vi "TLB Native Dynamic Events ver 0.26b.vi"() -> ()   [LabVIEW 2018] (continued)
      tunnel: [w2960 w2972 w2987 w3011 w3021 w3036 w3050 w3065 w3080 w3095 w3109 w3121 w3137 w3149 w3171 w3194 w3211 w3220 w3237 w3263 w3274 w3287 w3302 w3315 w3330 w3351 w3387 w3417 w3429 w3442 w3454 w3470 w3486 w3499 w3510 w3537 w3560 w3572 w3580 w3591 w3602 w3615 w3628 w3647 w3658 w3675 w3682 w3703 w3718 w3733 w3748 w3763 w3778 w3792] -> w237
      tunnel: w235 -> [w2958 w2971 w2988 w3012 w3022 w3037 w3051 w3064 w3081 w3096 w3108 w3120 w3136 w3148 w3168 w3195 w3212 w3219 w3234 w3260 w3273 w3286 w3301 w3314 w3329 w3349 w3385 w3415 w3428 w3441 w3453 w3469 w3485 w3498 w3509 w3538 w3561 w3573 w3579 w3590 w3601 w3614 w3627 w3648 w3659 w3676 w3681 w3697 w3712 w3727 w3742 w3757 w3772 w3786]
      tunnel: [w2958 w2971 w2988 w3012 w3022 w3037 w3051 w3064 w3081 w3096 w3108 w3120 w3136 w3148 w3168 w3195 w3212 w3219 w3234 w3260 w3273 w3286 w3301 w3314 w3328 w3348 w3384 w3415 w3428 w3441 w3453 w3469 w3485 w3498 w3509 w3538 w3561 w3573 w3579 w3590 w3601 w3614 w3627 w3648 w3659 w3676 w3681 w3697 w3710 w3725 w3740 w3755 w3770 w3785] -> w234
      tunnel: w232 -> [_ _ _ _ _ _ _ _ _ _ _ _ _ _ _ _ _ _ _ _ _ _ _ _ _ _ _ _ _ _ _ _ _ _ _ _ _ _ _ _ _ _ _ _ _ w3667 _ _ _ _ _ _ _ _]
      tunnel: [w2957 w2970 w2982 w3002 w3016 w3031 w3046 w3060 w3076 w3090 w3105 w3119 w3130 w3147 w3165 w3186 w3213 w3218 w3231 w3259 w3272 w3285 w3300 w3311 w3322 w3342 w3376 w3414 w3427 w3440 w3458 w3463 w3479 w3495 w3507 w3522 w3554 w3565 w3585 w3589 w3600 w3613 w3626 w3639 w3660 w3665 w3680 w3696 w3707 w3722 w3737 w3752 w3767 w3782] -> w228
      tunnel: w229 -> [w2957 w2970 w2982 w3002 w3016 w3031 w3046 w3060 w3076 w3090 w3105 w3119 w3130 w3147 w3165 w3187 w3213 w3218 w3231 w3259 w3272 w3285 w3300 w3311 w3322 w3343 w3377 w3414 w3427 w3440 w3458 w3463 w3479 w3495 w3507 w3522 w3554 w3565 w3585 w3589 w3600 w3613 w3626 w3639 w3660 w3665 w3680 w3696 w3707 w3722 w3737 w3752 w3767 w3782]
      tunnel: w226 -> [_ _ _ _ _ _ _ _ w3075 _ _ _ _ _ _ _ _ _ _ _ _ _ _ _ _ _ _ _ _ _ _ _ _ _ _ _ _ _ _ _ _ _ _ _ _ _ _ _ _ _ _ _ _ _]
      tunnel: w224 -> [w2956 w2969 w2981 w2996 w3015 w3030 w3045 w3059 w3073 w3089 w3104 w3118 w3129 w3146 w3164 w3182 w3206 w3217 w3229 w3258 w3271 w3284 w3299 w3310 w3325 w3345 w3380 w3413 w3426 w3439 w3450 w3462 w3478 w3494 w3506 w3519 w3553 w3564 w3576 w3588 w3599 w3612 w3625 w3638 w3651 w3664 w3679 w3695 w3706 w3721 w3736 w3751 w3766 w3781]
      tunnel: [w2956 w2969 w2981 w2996 w3015 w3030 w3045 w3059 w3073 w3089 w3104 w3118 w3129 w3146 w3164 w3182 w3205 w3217 w3229 w3258 w3271 w3284 w3299 w3310 w3324 w3344 w3379 w3413 w3426 w3439 w3450 w3462 w3478 w3494 w3506 w3519 w3553 w3564 w3576 w3588 w3599 w3612 w3625 w3638 w3651 w3664 w3679 w3695 w3706 w3721 w3736 w3751 w3766 w3781] -> w223
      tunnel: [_ _ _ _ _ _ _ _ _ _ _ _ _ _ _ _ _ _ _ _ _ _ _ _ _ _ _ _ _ _ _ _ _ _ _ w3518 w3548 _ _ _ _ _ _ _ _ _ _ _ _ _ _ _ _ _] -> w221
      tunnel: w219 -> [w2955 w2968 w2980 w2995 w3014 w3029 w3044 w3058 w3072 w3088 w3103 w3117 w3128 w3145 w3163 w3181 w3197 w3216 w3227 w3257 w3270 w3283 w3298 w3309 w3326 w3346 w3381 w3412 w3425 w3438 w3449 w3461 w3477 w3493 w3505 w3517 w3552 w3563 w3575 w3587 w3598 w3611 w3624 w3637 w3650 w3663 w3678 w3694 w3705 w3720 w3735 w3750 w3765 w3780]
      tunnel: [w2955 w2968 w2980 w2995 w3014 w3029 w3044 w3058 w3072 w3088 w3103 w3117 w3128 w3145 w3163 w3181 w3197 w3216 w3227 w3257 w3270 w3283 w3298 w3309 w3326 w3346 w3381 w3412 w3425 w3438 w3449 w3461 w3477 w3493 w3505 w3517 w3552 w3563 w3575 w3587 w3598 w3611 w3624 w3637 w3650 w3663 w3678 w3694 w3705 w3720 w3735 w3750 w3765 w3780] -> w218
      tunnel: w214 -> [w2954 w2967 w2979 w2994 w3013 w3028 w3043 w3057 w3071 w3087 w3102 w3116 w3127 w3144 w3162 w3178 w3196 w3215 w3226 w3256 w3269 w3282 w3297 w3308 w3321 w3339 w3374 w3411 w3424 w3437 w3448 w3460 w3476 w3492 w3504 w3516 w3546 w3562 w3574 w3586 w3597 w3610 w3623 w3636 w3649 w3662 w3677 w3693 w3704 w3719 w3734 w3749 w3764 w3779]
      tunnel: [w2954 w2967 w2979 w2994 w3013 w3028 w3043 w3057 w3071 w3087 w3102 w3116 w3127 w3144 w3162 w3178 w3196 w3215 w3226 w3256 w3269 w3282 w3297 w3308 w3321 w3339 w3374 w3411 w3424 w3437 w3448 w3460 w3476 w3492 w3504 w3516 w3539 w3562 w3574 w3586 w3597 w3610 w3623 w3636 w3649 w3662 w3677 w3693 w3704 w3719 w3734 w3749 w3764 w3779] -> w213
      frame "Exit" {
        # ">>State Logic  >>"
        # ">>> Time cluster >>>"
        # ">>> Yaw >>>"
        # ">>> Stepper position >>>"
        # ">>> Encoders >>>"
        # ">>> Object detection >>>"
        # ">>> Ultrasonic Sensors Detect >>>"
        n70 = call "Imaq Dispose"("All Images? (No)"=TRUE) -> ()  [unwired: 5 in, 1 out]
      }
      frame "----Movement States----" {
        # ">>State Logic  >>"
        # ">>> Time cluster >>>"
        # ">>> Yaw >>>"
        # ">>> Stepper position >>>"
        # ">>> Encoders >>>"
        # ">>> Object detection >>>"
        # ">>> Ultrasonic Sensors Detect >>>"
      }
      frame "FORWARD" {
        # ">>State Logic  >>"
        # ">>> Time cluster >>>"
        # ">>> Yaw >>>"
        # ">>> Stepper position >>>"
        # ">>> Encoders >>>"
        # ">>> Object detection >>>"
        # ">>> Ultrasonic Sensors Detect >>>"
        n71 = Unbundle By Name(w2987) -> ("Yaw"=w2983:dbl)
        n72 = call "MOTOR CONTROL WITH PID AE.vi"("Yaw"=w2983, "Speed"=50.0, "Direction"=MOTOR_CONTROL_WITH_PID_AE_DIRECTION_TYPE_DEF."y-axis movement", "AE Mode"=MOTOR_CONTROL_WITH_PID_AE_DATA_MODE_TYPE_DEF."Write to AE") -> ()  [unwired: 1 out]
      }
      frame "FORWARD - IR ASSIST" {
        # ">>State Logic  >>"
        # ">>> Time cluster >>>"
        # ">>> Yaw >>>"
        # ">>> Stepper position >>>"
        # ">>> Encoders >>>"
        # ">>> Object detection >>>"
        # ">>> Ultrasonic Sensors Detect >>>"
        n73 = Unbundle By Name(w3002) -> ("Left IR Sensor"=w3001:dbl)
        n74 = Subtract(x=w3001, y=10.0) -> (x-y=w2999:dbl)
        n75 = Multiply(x=w2999, y=0.2) -> (x*y=w2997:dbl)
        n76 = call "MOTOR CONTROL WITH PID AE.vi"("Yaw"=w2997, "Speed"=40.0, "Direction"=MOTOR_CONTROL_WITH_PID_AE_DIRECTION_TYPE_DEF."y-axis movement", "AE Mode"=MOTOR_CONTROL_WITH_PID_AE_DATA_MODE_TYPE_DEF."Write to AE") -> ()  [unwired: 1 out]
      }
      frame "LEFT" {
        # ">>State Logic  >>"
        # ">>> Time cluster >>>"
        # ">>> Yaw >>>"
        # ">>> Stepper position >>>"
        # ">>> Encoders >>>"
        # ">>> Object detection >>>"
        # ">>> Ultrasonic Sensors Detect >>>"
        n77 = Unbundle By Name(w3021) -> ("Yaw"=w3018:dbl)
        n78 = call "MOTOR CONTROL WITH PID AE.vi"("Yaw"=w3018, "Speed"=-20.0, "Direction"=MOTOR_CONTROL_WITH_PID_AE_DIRECTION_TYPE_DEF."x-axis movement", "AE Mode"=MOTOR_CONTROL_WITH_PID_AE_DATA_MODE_TYPE_DEF."Write to AE") -> ()  [unwired: 1 out]
      }
      frame "RIGHT" {
        # ">>> Time cluster >>>"
        # ">>> Yaw >>>"
        # ">>> Stepper position >>>"
        # ">>> Encoders >>>"
        # ">>> Object detection >>>"
        # ">>> Ultrasonic Sensors Detect >>>"
        n79 = Unbundle By Name(w3036) -> ("Yaw"=w3032:dbl)
        n80 = call "MOTOR CONTROL WITH PID AE.vi"("Yaw"=w3032, "Speed"=20.0, "Direction"=MOTOR_CONTROL_WITH_PID_AE_DIRECTION_TYPE_DEF."x-axis movement", "AE Mode"=MOTOR_CONTROL_WITH_PID_AE_DATA_MODE_TYPE_DEF."Write to AE") -> ()  [unwired: 1 out]
      }
      frame "R-ACW" {
        # ">>> IR Sensors >>>"
        # ">>> Time cluster >>>"
        # ">>> Yaw >>>"
        # ">>> Stepper position >>>"
        # ">>> Encoders >>>"
        # ">>> Object detection >>>"
        # ">>> Ultrasonic Sensors Detect >>>"
        n81 = call "MOTOR CONTROL WITH PID AE.vi"("Speed"=10.0, "Direction"=MOTOR_CONTROL_WITH_PID_AE_DIRECTION_TYPE_DEF."rotation", "AE Mode"=MOTOR_CONTROL_WITH_PID_AE_DATA_MODE_TYPE_DEF."Write to AE") -> ()  [unwired: 1 in, 1 out]
      }
      frame "R-CW" {
        (unwired) -0.2 ("Speed")
        # ">>> Time cluster >>>"
        # ">>> Yaw >>>"
        # ">>> Stepper position >>>"
        # ">>> Encoders >>>"
        # ">>> Object detection >>>"
        # ">>> Ultrasonic Sensors Detect >>>"
        n82 = call "MOTOR CONTROL WITH PID AE.vi"("Speed"=-10.0, "Direction"=MOTOR_CONTROL_WITH_PID_AE_DIRECTION_TYPE_DEF."rotation", "AE Mode"=MOTOR_CONTROL_WITH_PID_AE_DATA_MODE_TYPE_DEF."Write to AE") -> ()  [unwired: 1 in, 1 out]
      }
      frame "X AXIS - SLOW" {
        # ">>> Line Sensor Cluster>>>"
        # ">>> IR Sensors >>>"
        # ">>> Time cluster >>>"
        # ">>> Yaw >>>"
        # ">>> Stepper position >>>"
        # ">>> Encoders >>>"
        # ">>> Object detection >>>"
        # ">>> Ultrasonic Sensors Detect >>>"
        n83 = Unbundle By Name(w3075) -> ("xSpeed"=w3074:dbl)
        n84 = Unbundle By Name(w3080) -> ("Yaw"=w3077:dbl)
        n85 = call "MOTOR CONTROL WITH PID AE.vi"("Yaw"=w3077, "Speed"=w3074, "Direction"=MOTOR_CONTROL_WITH_PID_AE_DIRECTION_TYPE_DEF."x-axis movement", "AE Mode"=MOTOR_CONTROL_WITH_PID_AE_DATA_MODE_TYPE_DEF."Write to AE") -> ()  [unwired: 1 out]
      }
      frame "REVERSE" {
        # ">>> Time cluster >>>"
        # ">>> Yaw >>>"
        # ">>> Stepper position >>>"
        # ">>> Encoders >>>"
        # ">>> Object detection >>>"
        # ">>> Ultrasonic Sensors Detect >>>"
        n86 = Unbundle By Name(w3095) -> ("Yaw"=w3091:dbl)
        n87 = call "MOTOR CONTROL WITH PID AE.vi"("Yaw"=w3091, "Speed"=-50.0, "Direction"=MOTOR_CONTROL_WITH_PID_AE_DIRECTION_TYPE_DEF."y-axis movement", "AE Mode"=MOTOR_CONTROL_WITH_PID_AE_DATA_MODE_TYPE_DEF."Write to AE") -> ()  [unwired: 1 out]
      }
      frame "STOP" {
        n88 = Wait (ms)(milliseconds to wait=u32 100) -> ()  [unwired: 1 out]
        n89 = call "MOTOR CONTROL WITH PID AE.vi"("Direction"=MOTOR_CONTROL_WITH_PID_AE_DIRECTION_TYPE_DEF."stop", "AE Mode"=MOTOR_CONTROL_WITH_PID_AE_DATA_MODE_TYPE_DEF."Write to AE") -> ()  [unwired: 2 in, 1 out]
      }
      frame "----SENSOR READING---- " {
      }
      frame "READ ENCODERS" {
        # ">>> Time cluster >>>"
        # ">>> Yaw >>>"
        # ">>> Stepper position >>>"
        # ">>> Object detection >>>"
        # ">>> Current encoder distance >>>"
        # ">>> Ultrasonic Sensors Detect >>>"
        n90 = call "MOTOR CONTROL WITH PID AE.vi"("AE Mode"=MOTOR_CONTROL_WITH_PID_AE_DATA_MODE_TYPE_DEF."Read from AE") -> ("Speed & distance"=w3134:T15)  [unwired: 3 in]
        n91 = Unbundle By Name(w3134) -> ("xDistance"=w3133:dbl, "yDistance"=w3132:dbl, "wDistance"=w3131:dbl)
        n92 = Bundle By Name(cluster=w3141, "xDistance"=w3133, "yDistance"=w3132, "wDistance"=w3131) -> (w3140:T8)
      }
      frame "READ ULTRASONIC" {
        (unwired) navX_type_def."Read Values" ("Mode")
        (unwired) MOTOR_CONTROL_NO_PID_Type_Def."Latch" ("Direction")
        # ">>> Line Sensor Cluster>>>"
        # ">>> IR Sensors >>>"
        # ">>State Logic  >>"
        # ">>> Time cluster >>>"
        # ">>> Ultrasonic Sensors Detect >>>"
        # ">>> Object detection >>>"
        # ">>> Encoders >>>"
        # ">>> Stepper position >>>"
        # ">>> Yaw >>>"
        n93 = call "Arduino Interfacing VI.vi"("AE Mode"=Arduino_Interfacing."Read From Arduino") -> ("Arduino Data"=w3154:T17)  [unwired: 3 in, 1 out]
        n94 = Unbundle By Name(w3154) -> ("PING A"=w3153:u8, "PING B"=w3152:u8, "PING C"=w3151:u8, "PING D"=w3150:u8)
        n95 = Bundle By Name(cluster=w3160, "PING_A"=w3153, "PING_B"=w3152, "PING_C"=w3151, "PING_D"=w3150) -> (w3161:T9)
      }
      frame "READ NAVX" {
        # ">> Item Selection Bias >>"
        # ">>State Logic  >>"
        # ">>> Line Sensor Cluster>>>"
        # ">>> IR Sensors >>>"
        # ">>> Time cluster >>>"
        # ">>> Yaw >>>"
        # ">>> Ultrasonic Sensors Detect >>>"
        # ">>> Object detection >>>"
        # ">>> Encoders >>>"
        # ">>> Stepper position >>>"
        n96 = call "navX reading VI.vi"("Mode"=navX_type_def."Read Values") -> ("NavX Readings"=w3167:T16)  [unwired: 2 in, 3 out]
        n97 = Unbundle By Name(w3167) -> ("Heading"=w3166:dbl)
        n98 = Unbundle By Name(w3167) -> ("Yaw"=w3170:dbl)
        n99 = Bundle By Name(cluster=w3172, "Yaw"=w3170, "Compass"=w3166) -> (w3171:T6)
      }
      frame "READ IR" {
        w3180 = T42 [enum."B/AI2"] items=["Not Connected", "AudioIn/Left", "AudioIn/Right", "C/AI0", "C/AI1", "A/AI0", "A/AI1", "A/AI2", "A/AI3", "A/AI4", "A/AI5", "A/AI6", "A/AI7", "B/AI0", "B/AI1", "B/AI2", "B/AI3", "B/AI4", "B/AI5", "B/AI6", "B/AI7", "AI/AI0", "AI/AI1", "AI/AI2", "AI/AI3", "A/AI0 (DIFF)", "A/AI1 (DIFF)", "A/AI2 (DIFF)", "A/AI3 (DIFF)", "B/AI0 (DIFF)", "B/AI1 (DIFF)", "B/AI2 (DIFF)", "B/AI3 (DIFF)"] ("AI Channel")
        w3184 = T42 [enum."B/AI1"] items=["Not Connected", "AudioIn/Left", "AudioIn/Right", "C/AI0", "C/AI1", "A/AI0", "A/AI1", "A/AI2", "A/AI3", "A/AI4", "A/AI5", "A/AI6", "A/AI7", "B/AI0", "B/AI1", "B/AI2", "B/AI3", "B/AI4", "B/AI5", "B/AI6", "B/AI7", "AI/AI0", "AI/AI1", "AI/AI2", "AI/AI3", "A/AI0 (DIFF)", "A/AI1 (DIFF)", "A/AI2 (DIFF)", "A/AI3 (DIFF)", "B/AI0 (DIFF)", "B/AI1 (DIFF)", "B/AI2 (DIFF)", "B/AI3 (DIFF)"] ("AI Channel")
        w3189 = T42 [enum."B/AI0"] items=["Not Connected", "AudioIn/Left", "AudioIn/Right", "C/AI0", "C/AI1", "A/AI0", "A/AI1", "A/AI2", "A/AI3", "A/AI4", "A/AI5", "A/AI6", "A/AI7", "B/AI0", "B/AI1", "B/AI2", "B/AI3", "B/AI4", "B/AI5", "B/AI6", "B/AI7", "AI/AI0", "AI/AI1", "AI/AI2", "AI/AI3", "A/AI0 (DIFF)", "A/AI1 (DIFF)", "A/AI2 (DIFF)", "A/AI3 (DIFF)", "B/AI0 (DIFF)", "B/AI1 (DIFF)", "B/AI2 (DIFF)", "B/AI3 (DIFF)"] ("AI Channel")
        # ">>> Line Sensor Cluster>>>"
        # ">>> IR Sensors >>>"
        # ">>State Logic  >>"
        # ">>> Time cluster >>>"
        # ">>> Ultrasonic Sensors Detect >>>"
        # ">>> Object detection >>>"
        # ">>> Encoders >>>"
        # ">>> Stepper position >>>"
        # ">>> Yaw >>>"
        n100 = call <vilib>:"Sharp IR.vi"("AI Channel"=w3189) -> ("Sharp IR Distance"=w3185:dbl)  [unwired: 8 in, 2 out]
        n101 = call <vilib>:"Sharp IR.vi"("AI Channel"=w3184) -> ("Sharp IR Distance"=w3183:dbl)  [unwired: 8 in, 2 out]
        n102 = call <vilib>:"Sharp IR.vi"("AI Channel"=w3180) -> ("Sharp IR Distance"=w3179:dbl)  [unwired: 8 in, 2 out]
        n103 = Bundle By Name(cluster=w3187, "Left IR Sensor"=w3185, "Arm IR Sensor"=w3183, "Bottom IR Sensor"=w3179) -> (w3186:T5)
      }
      frame "READ LINE SENSOR" {
        # ">>> IR Sensors >>>"
        # ">>> Line Sensor Cluster>>>"
        # ">>State Logic  >>"
        # ">>> Time cluster >>>"
        # ">>> Object detection >>>"
        # ">>> Yaw >>>"
        # ">>> Ultrasonic Sensors Detect >>>"
        # ">>> Encoders >>>"
        # ">>> Stepper position >>>"
        n104 = call "Line Sensor AE.vi"("AE State"=Line_Sensor_AE_Type_Def."READ FROM LINE SENSORS") -> ("Line Detected?"=w3203:bool, "Line Sensor Raw Values"=w3202:T44)
        n105 = Unbundle By Name(w3202) -> ("S1"=w3201:dbl, "S2"=w3200:dbl, "S3"=w3199:dbl, "S4"=w3198:dbl)
        n106 = Bundle By Name(cluster=w3206, "Line Detected?"=w3203, "S1"=w3201, "S2"=w3200, "S3"=w3199, "S4"=w3198) -> (w3205:T4)
      }
      frame "----SYSTEM MODES----" {
        (unwired) I2C_MASTER_Type_Def."Last State" ("Arduino Mode")
        # ">>> Object detection >>>"
        # ">>> Yaw >>>"
        # ">>> Ultrasonic Sensors Detect >>>"
        # ">>> Encoders >>>"
        # ">>> Stepper position >>>"
      }
      frame "INIT" {
        w3249 = u8 0
        w3250 = 0.0
        # ">>> IR Sensors >>>"
        # ">>> IR Sensors >>>"
        # ">>> Line Sensor Cluster>>>"
        # ">>> Time cluster >>>"
        # ">>> Object detection >>>"
        # ">>> Yaw >>>"
        # ">>> Ultrasonic Sensors Detect >>>"
        # ">>> Encoders >>>"
        # ">>> Stepper position >>>"
        # ">>State Logic  >>"
        n107 = call "Arduino Interfacing VI.vi"("AE Mode"=Arduino_Interfacing."Initialize") -> ()  [unwired: 3 in, 2 out]
        n108 = call "FGV Stop.vi"("Init/Read/Write State"=States_for_Action_Engine."Initialize") -> ()  [unwired: 2 in, 2 out]
        n109 = call "Elasped Timer.vi"("Action"=Elapsed_timer_control."Initialize") -> ()  [unwired: 7 in, 4 out]
        n110 = call "MOTOR CONTROL WITH PID AE.vi"("AE Mode"=MOTOR_CONTROL_WITH_PID_AE_DATA_MODE_TYPE_DEF."Init AE") -> ()  [unwired: 3 in, 1 out]
        n111 = call "IMAQ Reference AE.vi"("IMAQ AE States"=IMAQ_Reference_AE."Initialize AE") -> ()  [unwired: 1 in, 2 out]
        n112 = call "Line Sensor AE.vi"("AE State"=Line_Sensor_AE_Type_Def."INIT AE") -> ()  [unwired: 2 out]
        n113 = Bundle By Name(cluster=w3243, "Recognized Object"=FALSE, "Object X coordinate"=0.0, "Object Y coordinate"=0.0) -> (w3242:T11)
        n114 = Bundle By Name(cluster=w3248, "y Stepper Position"=u8 0, "z Stepper Position"=u8 0) -> (w3247:T7)
        n115 = Bundle By Name(cluster=w3252, "xDistance"=w3250, "yDistance"=w3250, "wDistance"=w3250) -> (w3251:T8)
        n116 = Bundle By Name(cluster=w3254, "PING_A"=w3249, "PING_B"=w3249, "PING_C"=w3249, "PING_D"=w3249) -> (w3255:T9)
        n117 = Bundle By Name(cluster=w3238, "Yaw"=0.0) -> (w3237:T6)
      }
      frame "ARDUINO - ULTRASONIC" {
        # ">>> Time cluster >>>"
        # ">>> Line Sensor Cluster>>>"
        # ">>> Object detection >>>"
        # ">>> Yaw >>>"
        # ">>> Ultrasonic Sensors Detect >>>"
        # ">>> Encoders >>>"
        # ">>> Stepper position >>>"
        # ">>State Logic  >>"
        n118 = call "Arduino Interfacing VI.vi"("Data to Write"=I2C_MASTER_WRITE_NEW_Type_Def."Ultrasonic sensors", "AE Mode"=Arduino_Interfacing."Write to Arduino") -> ()  [unwired: 2 in, 2 out]
      }
      frame "NAVX CALIBRATE" {
        # ">>> Object detection >>>"
        # ">>> Yaw >>>"
        # ">>> Ultrasonic Sensors Detect >>>"
        # ">>> Encoders >>>"
        # ">>> Stepper position >>>"
        # ">>State Logic  >>"
        # "Adds a 15 second delay to the startup process \nfor the NavX to calibrate"
        n119 = Wait (ms)(milliseconds to wait=u32 1000) -> ()  [unwired: 1 out]
      }
      frame "NO ACTION", Default {
        (unwired) u8 0 ("y Stepper value")
        (unwired) TRUE ("Latch")
        (unwired) navX_type_def."Read Values" ("Mode")
        (unwired) MOTOR_CONTROL_NO_PID_Type_Def."Latch" ("Direction")
        # ">>> Object detection >>>"
        # ">>> Yaw >>>"
        # ">>> Ultrasonic Sensors Detect >>>"
        # ">>> Encoders >>>"
        # ">>> Stepper position >>>"
        # ">>State Logic  >>"
        n120 = case shown="4" w3291 {
          tunnel: [0 100] -> w3293
          frame 1, Default {
          }
          frame 4 {
          }
        }
      }
      frame "----RESET CASES----" {
        (unwired) I2C_MASTER_Type_Def."Last State" ("Arduino Mode")
        # ">>> Object detection >>>"
        # ">>> Yaw >>>"
        # ">>> Ultrasonic Sensors Detect >>>"
        # ">>> Encoders >>>"
        # ">>> Stepper position >>>"
        # ">>State Logic  >>"
      }
      frame "RESET ENCODERS" {
        # ">>> Object detection >>>"
        # ">>> Yaw >>>"
        # ">>> Ultrasonic Sensors Detect >>>"
        # ">>> Encoders >>>"
        # ">>> Stepper position >>>"
        # ">>State Logic  >>"
        n121 = call "MOTOR CONTROL WITH PID AE.vi"("Direction"=MOTOR_CONTROL_WITH_PID_AE_DIRECTION_TYPE_DEF."reset encoders", "AE Mode"=MOTOR_CONTROL_WITH_PID_AE_DATA_MODE_TYPE_DEF."Write to AE") -> ()  [unwired: 2 in, 1 out]
      }
      frame "RESET FLAGS" {
        # ">>> Line Sensor Cluster>>>"
        # ">>> IR Sensors >>>"
        # ">>> Time cluster >>>"
        # ">>> Object detection >>>"
        # ">>> Yaw >>>"
        # ">>> Ultrasonic Sensors Detect >>>"
        # ">>> Encoders >>>"
        # ">>> Stepper position >>>"
        # ">>> Line Sensor Cluster>>>"
        # ">>> IR Sensors >>>"
        # ">>> Time cluster >>>"
        # ">>> Object detection >>>"
        # ">>> Yaw >>>"
        # ">>> Ultrasonic Sensors Detect >>>"
        # ">>> Encoders >>>"
        # ">>> Stepper position >>>"
        # "Resets BOOLEAN FLAGS only"
        n122 = Wait (ms)(milliseconds to wait=u32 20) -> ()  [unwired: 1 out]
        n123 = Bundle By Name(cluster=w3335, "Recognized Object"=FALSE) -> (w3334:T11)
        n124 = Bundle By Name(cluster=w3325, "Line Detected?"=FALSE) -> (w3324:T4)
        n125 = Bundle By Name(cluster=w3329, "Time up flag"=FALSE) -> (w3328:T3)
      }
      frame "RESET SENSOR VALUES" {
        w3340 = 0.0 ("S4")
        w3341 = 0.0 ("S4")
        # "Resets SENSOR VALUES only"
        # ">>> Line Sensor Cluster>>>"
        # ">>> IR Sensors >>>"
        # ">>> Time cluster >>>"
        # ">>> Object detection >>>"
        # ">>> Yaw >>>"
        # ">>> Ultrasonic Sensors Detect >>>"
        # ">>> Encoders >>>"
        # ">>> Stepper position >>>"
        # ">>> Line Sensor Cluster>>>"
        # ">>> IR Sensors >>>"
        # ">>> Time cluster >>>"
        # ">>> Object detection >>>"
        # ">>> Yaw >>>"
        # ">>> Ultrasonic Sensors Detect >>>"
        # ">>> Encoders >>>"
        # ">>> Stepper position >>>"
        # "Resets any software variables\nand/or non-critical states"
        n126 = Wait (ms)(milliseconds to wait=u32 20) -> ()  [unwired: 1 out]
        n127 = Bundle By Name(cluster=w3349, "SET TIME TO CHECK"=0.0) -> (w3348:T3)
        n128 = Bundle By Name(cluster=w3365, "Object X coordinate"=0.0, "Object Y coordinate"=0.0) -> (w3364:T11)
        n129 = Bundle By Name(cluster=w3356, "y Stepper Position"=u8 0, "z Stepper Position"=u8 0) -> (w3355:T7)
        n130 = Bundle By Name(cluster=w3343, "Left IR Sensor"=w3340, "Arm IR Sensor"=w3340) -> (w3342:T5)
        n131 = Bundle By Name(cluster=w3361, "xDistance"=0.0, "yDistance"=0.0, "wDistance"=0.0) -> (w3360:T8)
        n132 = Bundle By Name(cluster=w3372, "PING_A"=u8 0, "PING_B"=u8 0, "PING_C"=u8 0, "PING_D"=u8 0) -> (w3371:T9)
        n133 = Bundle By Name(cluster=w3352, "Yaw"=0.0) -> (w3351:T6)
        n134 = Bundle By Name(cluster=w3345, "S1"=w3341, "S2"=w3341, "S3"=w3341, "S4"=w3341) -> (w3344:T4)
      }
      frame "RESET ALL SENSORS" {
        w3375 = 0.0 ("SET TIME TO CHECK")
        # ">>> Line Sensor Cluster>>>"
        # ">>> IR Sensors >>>"
        # ">>> Time cluster >>>"
        # ">>> Object detection >>>"
        # ">>> Yaw >>>"
        # ">>> Ultrasonic Sensors Detect >>>"
        # ">>> Encoders >>>"
        # ">>> Stepper position >>>"
        # ">>> Line Sensor Cluster>>>"
        # ">>> IR Sensors >>>"
        # ">>> Time cluster >>>"
        # ">>> Object detection >>>"
        # ">>> Yaw >>>"
        # ">>> Ultrasonic Sensors Detect >>>"
        # ">>> Encoders >>>"
        # ">>> Stepper position >>>"
        # "Resets ALL SENSOR PARAMTERS"
        n135 = Wait (ms)(milliseconds to wait=u32 20) -> ()  [unwired: 1 out]
        n136 = Bundle By Name(cluster=w3385, "Time up flag"=FALSE, "SET TIME TO CHECK"=0.0) -> (w3384:T3)
        n137 = Bundle By Name(cluster=w3402, "Recognized Object"=FALSE, "Object X coordinate"=0.0, "Object Y coordinate"=0.0) -> (w3401:T11)
        n138 = Bundle By Name(cluster=w3392, "y Stepper Position"=u8 0, "z Stepper Position"=u8 0) -> (w3391:T7)
        n139 = Bundle By Name(cluster=w3380, "Line Detected?"=FALSE) -> (w3379:T4)
        n140 = Bundle By Name(cluster=w3377, "Left IR Sensor"=w3375, "Arm IR Sensor"=w3375) -> (w3376:T5)
        n141 = Bundle By Name(cluster=w3397, "xDistance"=0.0, "yDistance"=0.0, "wDistance"=0.0) -> (w3396:T8)
        n142 = Bundle By Name(cluster=w3409, "PING_A"=u8 0, "PING_B"=u8 0, "PING_C"=u8 0, "PING_D"=u8 0) -> (w3408:T9)
        n143 = Bundle By Name(cluster=w3388, "Yaw"=0.0) -> (w3387:T6)
      }
      frame "RESET YAW" {
        n144 = Wait (ms)(milliseconds to wait=u32 100) -> ()  [unwired: 1 out]
        n145 = call "navX reading VI.vi"("Mode"=navX_type_def."Zero Yaw") -> ()  [unwired: 2 in, 4 out]
      }
      frame "RESET ARM" {
        n146 = call "Arduino Interfacing VI.vi"("Data to Write"=I2C_MASTER_WRITE_NEW_Type_Def."Soft Reset", "AE Mode"=Arduino_Interfacing."Write to Arduino") -> ()  [unwired: 2 in, 2 out]
      }
      frame "--------CAM STATES-------" {
      }
      frame "OPEN IMAQ REF" {
        # ">>> Line Sensor Cluster>>>"
        # ">>State Logic  >>"
        # ">>> Time cluster >>>"
        # ">>> Object detection >>>"
        # ">>> Yaw >>>"
        # ">>> Ultrasonic Sensors Detect >>>"
        # ">>> Encoders >>>"
        # ">>> Stepper position >>>"
        # ">>> IR Sensors >>>"
        n147 = call "IMAQ Reference AE.vi"("IMAQ AE States"=IMAQ_Reference_AE."Initialize AE") -> ()  [unwired: 1 in, 2 out]
      }
      frame "OPEN LOG CAM" {
        n148 = call "Webcam AE.vi"("Session In"=T40 "cam0", "Camera states"=Webcam_AE."Initialize Camera") -> ("error out"=w3466:errorcluster, "Session Out"=w3465:T40)  [unwired: 1 in, 1 out]
        n149 = call "Webcam AE.vi"("error in (no error)"=w3466, "Session In"=w3465, "Camera states"=Webcam_AE."Open Camera") -> ()  [unwired: 3 out]
      }
      frame "OPEN LIFE CAM" {
        n150 = call "Webcam AE.vi"("Session In"=T40 "cam1", "Camera states"=Webcam_AE."Initialize Camera") -> ("error out"=w3482:errorcluster, "Session Out"=w3481:T40)  [unwired: 1 in, 1 out]
        n151 = call "Webcam AE.vi"("error in (no error)"=w3482, "Session In"=w3481, "Camera states"=Webcam_AE."Open Camera") -> ()  [unwired: 3 out]
      }
      frame "CAM ACQ" {
        # ">>State Logic  >>"
        # ">>> Time cluster >>>"
        # ">>> Yaw >>>"
        # ">>> Stepper position >>>"
        # ">>> Encoders >>>"
        # ">>> Object detection >>>"
        # ">>> Ultrasonic Sensors Detect >>>"
        n152 = call "Webcam AE.vi"("Camera states"=Webcam_AE."Continuous Acquisition") -> ()  [unwired: 2 in, 3 out]
      }
      frame "CAM CLOSE" {
        # ">>State Logic  >>"
        # ">>> Time cluster >>>"
        # ">>> Yaw >>>"
        # ">>> Stepper position >>>"
        # ">>> Encoders >>>"
        # ">>> Object detection >>>"
        # ">>> Ultrasonic Sensors Detect >>>"
        n153 = call "Webcam AE.vi"("Camera states"=Webcam_AE."Close Camera") -> ()  [unwired: 2 in, 3 out]
      }
      frame "PROCESS IMAGE" {
        # ">>> Line Sensor Cluster>>>"
        # ">>> IR Sensors >>>"
        # ">> Item Selection Bias >>"
        # ">> Item Selection Bias >>"
        # ">>State Logic  >>"
        # ">>> Time cluster >>>"
        # ">>> Yaw >>>"
        # ">>> Stepper position >>>"
        # ">>> Encoders >>>"
        # ">>> Object detection >>>"
        # ">>> Ultrasonic Sensors Detect >>>"
        n154 = call "Webcam AE.vi"("Camera states"=Webcam_AE."Retrieve Image") -> ("error out"=w3530:errorcluster, "Image Out"=w3531:T46)  [unwired: 2 in, 1 out]
        n155 = call "IMAQ Reference AE.vi"("IMAQ AE States"=IMAQ_Reference_AE."Get IMAQ Reference") -> ("Image Out"=w3520:T46)  [unwired: 1 in, 1 out]
        n156 = call "Object Detection SubVI.vi"("Error In"=w3530, "Mode"=w3517, "Image Dest"=w3520, "Image in"=w3531) -> ("Error out"=w3518:errorcluster, "Object Center Coordinates"=w3527:cluster{"x":sgl, "y":sgl}, "Object detection cluster"=w3523:T47)  [unwired: 1 out]
        n157 = Unbundle By Name(w3523) -> ("Object detected?"=w3524:bool)
        n158 = Unbundle By Name(w3527) -> ("x"=w3526:sgl, "y"=w3525:sgl)
        n159 = Bundle By Name(cluster=w3529, "Recognized Object"=w3524, "Object X coordinate"=w3526, "Object Y coordinate"=w3525) -> (w3528:T11)
      }
      frame "COLOUR PROCESSING" {
        # ">>> Box Colour Detection >>>"
        # ">>> Box Colour Detection >>>"
        # ">>> Line Sensor Cluster>>>"
        # ">>> IR Sensors >>>"
        # ">> Item Selection Bias >>"
        # ">> Item Selection Bias >>"
        # ">>State Logic  >>"
        # ">>> Time cluster >>>"
        # ">>> Yaw >>>"
        # ">>> Stepper position >>>"
        # ">>> Encoders >>>"
        # ">>> Object detection >>>"
        # ">>> Ultrasonic Sensors Detect >>>"
        n160 = call "Webcam AE.vi"("Camera states"=Webcam_AE."Retrieve Image") -> ("error out"=w3549:errorcluster, "Image Out"=w3550:T46)  [unwired: 2 in, 1 out]
        n161 = call "Box Colour Detection SubVI.vi"("Image In"=w3550, "Error In"=w3549) -> ("Colour output boolean cluster"=w3547:T48, "Error out"=w3548:errorcluster)  [unwired: 1 out]
        n162 = Unbundle By Name(w3547) -> ("Red"=w3545:bool, "Black"=w3544:bool, "Blue"=w3543:bool, "Yellow"=w3542:bool, "Green"=w3541:bool, "No recognizable coolour"=w3540:bool)
        n163 = Bundle By Name(cluster=w3546, "Red"=w3545, "Black"=w3544, "Blue"=w3543, "Yellow"=w3542, "Green"=w3541, "Unknown"=w3540) -> (w3539:T1)
      }
      frame "DISPOSE CAM BUFFERS" {
        # ">> Item Selection Bias >>"
        # ">>> Line Sensor Cluster>>>"
        # ">>> IR Sensors >>>"
        # ">>State Logic  >>"
        # ">>> Time cluster >>>"
        # ">>> Yaw >>>"
        # ">>> Stepper position >>>"
        # ">>> Encoders >>>"
        # ">>> Object detection >>>"
        # ">>> Ultrasonic Sensors Detect >>>"
        n164 = call "Webcam AE.vi"("Camera states"=Webcam_AE."Dispose Camera Image Buffer") -> ()  [unwired: 2 in, 3 out]
      }
      frame "DISPOSE PROC BUFFERS" {
        # ">>> Line Sensor Cluster>>>"
        # ">>State Logic  >>"
        # ">>> IR Sensors >>>"
        # ">>> Time cluster >>>"
        # ">>> Object detection >>>"
        # ">>> Yaw >>>"
        # ">>> Ultrasonic Sensors Detect >>>"
        # ">>> Encoders >>>"
        # ">>> Stepper position >>>"
        n165 = call "IMAQ Reference AE.vi"("IMAQ AE States"=IMAQ_Reference_AE."Dispose Processing Buffer") -> ()  [unwired: 1 in, 2 out]
      }
      frame "-----ARM ACTIONS-----" {
      }
      frame "CLOSE CLAW" {
        n166 = call "Arduino Interfacing VI.vi"("Data to Write"=I2C_MASTER_WRITE_NEW_Type_Def."Close Claw", "AE Mode"=Arduino_Interfacing."Write to Arduino") -> ()  [unwired: 2 in, 2 out]
      }
      frame "OPEN CLAW" {
        n167 = call "Arduino Interfacing VI.vi"("Data to Write"=I2C_MASTER_WRITE_NEW_Type_Def."Open Claw", "AE Mode"=Arduino_Interfacing."Write to Arduino") -> ()  [unwired: 2 in, 2 out]
      }
      frame "Z STEPPER CAM HEIGHT" {
        n168 = call "Arduino Interfacing VI.vi"("Data to Write"=I2C_MASTER_WRITE_NEW_Type_Def."zStepper 6k", "AE Mode"=Arduino_Interfacing."Write to Arduino") -> ()  [unwired: 2 in, 2 out]
      }
      frame "Z STEPPER GRAB HEIGHT" {
        # ">>State Logic  >>"
        # ">>> Time cluster >>>"
        # ">>> Yaw >>>"
        # ">>> Stepper position >>>"
        # ">>> Encoders >>>"
        # ">>> Object detection >>>"
        # ">>> Ultrasonic Sensors Detect >>>"
        n169 = call "Arduino Interfacing VI.vi"("Data to Write"=I2C_MASTER_WRITE_NEW_Type_Def."zStepper 100", "AE Mode"=Arduino_Interfacing."Write to Arduino") -> ()  [unwired: 2 in, 2 out]
      }
      frame "Z STEPPER BOX HEIGHT" {
        # ">>> IR Sensors >>>"
        # ">>> Time cluster >>>"
        # ">>> Yaw >>>"
        # ">>> Stepper position >>>"
        # ">>> Encoders >>>"
        # ">>> Object detection >>>"
        # ">>> Ultrasonic Sensors Detect >>>"
        n170 = call "Arduino Interfacing VI.vi"("Data to Write"=I2C_MASTER_WRITE_NEW_Type_Def."zStepper 5k", "AE Mode"=Arduino_Interfacing."Write to Arduino") -> ()  [unwired: 2 in, 2 out]
      }
      frame "Y STEPPER CONTROL" {
        # ">>State Logic  >>"
        # ">>> yStepper command>>>"
        # ">>> Time cluster >>>"
        # ">>> Yaw >>>"
        # ">>> Stepper position >>>"
        # ">>> Encoders >>>"
        # ">>> Object detection >>>"
        # ">>> Ultrasonic Sensors Detect >>>"
        n171 = Unbundle By Name(w3667) -> ("yStepper desired"=w3666:u8)
        n172 = call "Arduino Interfacing VI.vi"("y Stepper value"=w3666, "Data to Write"=I2C_MASTER_WRITE_NEW_Type_Def."yStepper control", "AE Mode"=Arduino_Interfacing."Write to Arduino") -> ()  [unwired: 1 in, 2 out]
      }
      frame "READ STEPPER VALUES" {
        # ">>State Logic  >>"
        # ">>> Time cluster >>>"
        # ">>> Yaw >>>"
        # ">>> Stepper position >>>"
        # ">>> Encoders >>>"
        # ">>> Object detection >>>"
        # ">>> Ultrasonic Sensors Detect >>>"
        n173 = call "Arduino Interfacing VI.vi"("AE Mode"=Arduino_Interfacing."Read From Arduino") -> ("Arduino Data"=w3685:T17)  [unwired: 3 in, 1 out]
        n174 = Unbundle By Name(w3685) -> ("y Stepper Position"=w3684:u8, "z Stepper Position"=w3683:u8)
        n175 = Bundle By Name(cluster=w3688, "y Stepper Position"=w3684, "z Stepper Position"=w3683) -> (w3687:T7)
      }
      frame " -----TIMING-----" {
        # ">>State Logic  >>"
        # ">>> Time cluster >>>"
        # ">>> Yaw >>>"
        # ">>> Stepper position >>>"
        # ">>> Encoders >>>"
        # ">>> Object detection >>>"
        # ">>> Ultrasonic Sensors Detect >>>"
      }
      frame "SET TIMER 1" {
        # ">>State Logic  >>"
        # ">>> Time cluster >>>"
        # ">>> Yaw >>>"
        # ">>> Stepper position >>>"
        # ">>> Encoders >>>"
        # ">>> Object detection >>>"
        # ">>> Ultrasonic Sensors Detect >>>"
        n176 = call "Elasped Timer.vi"("Time Setting"=1.0, "Action"=Elapsed_timer_control."Initialize") -> ()  [unwired: 6 in, 4 out]
        n177 = Bundle By Name(cluster=w3712, "Time up flag"=FALSE) -> (w3710:T3)
      }
      frame "SET TIMER 2" {
        # ">>State Logic  >>"
        # ">>> Time cluster >>>"
        # ">>> Yaw >>>"
        # ">>> Stepper position >>>"
        # ">>> Encoders >>>"
        # ">>> Object detection >>>"
        # ">>> Ultrasonic Sensors Detect >>>"
        n178 = call "Elasped Timer.vi"("Time Setting"=2.0, "Action"=Elapsed_timer_control."Initialize") -> ()  [unwired: 6 in, 4 out]
        n179 = Bundle By Name(cluster=w3727, "Time up flag"=FALSE) -> (w3725:T3)
      }
      frame "SET TIMER 3" {
        # ">>State Logic  >>"
        # ">>> Time cluster >>>"
        # ">>> Yaw >>>"
        # ">>> Stepper position >>>"
        # ">>> Encoders >>>"
        # ">>> Object detection >>>"
        # ">>> Ultrasonic Sensors Detect >>>"
        n180 = call "Elasped Timer.vi"("Time Setting"=3.0, "Action"=Elapsed_timer_control."Initialize") -> ()  [unwired: 6 in, 4 out]
        n181 = Bundle By Name(cluster=w3742, "Time up flag"=FALSE) -> (w3740:T3)
      }
      frame "SET TIMER 4" {
        # ">>State Logic  >>"
        # ">>> Time cluster >>>"
        # ">>> Yaw >>>"
        # ">>> Stepper position >>>"
        # ">>> Encoders >>>"
        # ">>> Object detection >>>"
        # ">>> Ultrasonic Sensors Detect >>>"
        n182 = call "Elasped Timer.vi"("Time Setting"=4.0, "Action"=Elapsed_timer_control."Initialize") -> ()  [unwired: 6 in, 4 out]
        n183 = Bundle By Name(cluster=w3757, "Time up flag"=FALSE) -> (w3755:T3)
      }
      frame "SET TIMER 5" {
        # ">>State Logic  >>"
        # ">>> Time cluster >>>"
        # ">>> Yaw >>>"
        # ">>> Stepper position >>>"
        # ">>> Encoders >>>"
        # ">>> Object detection >>>"
        # ">>> Ultrasonic Sensors Detect >>>"
        n184 = call "Elasped Timer.vi"("Time Setting"=5.0, "Action"=Elapsed_timer_control."Initialize") -> ()  [unwired: 6 in, 4 out]
        n185 = Bundle By Name(cluster=w3772, "Time up flag"=FALSE) -> (w3770:T3)
      }
      frame "START TIMER" {
        # ">>State Logic  >>"
        # ">>> Time cluster >>>"
        # ">>> Yaw >>>"
        # ">>> Stepper position >>>"
        # ">>> Encoders >>>"
        # ">>> Object detection >>>"
        # ">>> Ultrasonic Sensors Detect >>>"
        n186 = call "Elasped Timer.vi"("Action"=Elapsed_timer_control."Start") -> ("Time Out?!"=w3783:bool)  [unwired: 7 in, 3 out]
        n187 = Bundle By Name(cluster=w3786, "Time up flag"=w3783) -> (w3785:T3)
      }
    }
    "State Logic" <- w254
    "Image Processing Error" <- w221
    n188 = local read "TASK ENABLE"() -> (w248:bool)
    n189 = Not(x=w248) -> (.not. x?=w247:bool)
    n190 = case shown="True" w255 {
      tunnel: w212 -> [w286 w331]
      tunnel: w262 -> [w282 w333]
      tunnel: [w286 w331] -> w267
      tunnel: [w282 w334] -> w266
      tunnel: w263 -> [_ w329]
      tunnel: w265 -> [_ w330]
      tunnel: w260 -> [w285 w336]
      tunnel: [w285 w336] -> w259
      tunnel: "STOP TASK" -> [_ w319]
      tunnel: w254 -> [w284 w335]
      tunnel: [w284 w332] -> w253
      tunnel: w250 -> [w283 w325]
      tunnel: [w283 w325] -> w249
      tunnel: w247 -> [_ w320]
      tunnel: [w281 w317] -> w246
      tunnel: w245 -> [w281 w316]
      tunnel: w243 -> [w280 w313]
      tunnel: [w280 w313] -> w242
      tunnel: w240 -> [w279 w309]
      tunnel: [w279 w309] -> w239
      tunnel: w237 -> [w278 w307]
      tunnel: [w278 w307] -> w236
      tunnel: w234 -> [w277 w305]
      tunnel: [w277 w305] -> w233
      tunnel: w232 -> [w276 w304]
      tunnel: [w276 w303] -> w231
      tunnel: [_ w301] -> w230
      tunnel: w228 -> [w275 w299]
      tunnel: [w275 w299] -> w227
      tunnel: w226 -> [w274 w298]
      tunnel: [w274 w297] -> w225
      tunnel: w223 -> [w273 w294]
      tunnel: [w273 w294] -> w222
      tunnel: [w272 w293] -> w220
      tunnel: w218 -> [w272 w292]
      tunnel: [_ w290] -> w217
      tunnel: [_ w289] -> w216
      tunnel: [_ w288] -> w215
      tunnel: w213 -> [w271 w287]
      tunnel: [w271 w287] -> w211
      frame False {
        # ">>> Box Colour Detection >>>"
        # ">>> Line Sensor Cluster>>>"
        # ">> Item Selection Bias >>"
        # ">>State Logic Queue Reference >>"
        # ">>Action states Queue Reference >>"
        # ">>True Stop Next State >>"
        # ">>State Logic  >>"
        # ">>> IR Sensors >>>"
        # ">>> Line Sensor Cluster>>>"
        # ">>> Line Sensor Cluster>>>"
        # ">>> Motor control cluster >>>"
        # ">>> yStepper command>>>"
        # ">>> Motor control cluster >>>"
        # ">>> yStepper command>>>"
        # ">>> Motor control cluster >>>"
        # ">>> IR Sensors >>>"
        # ">>> IR Sensors >>>"
        # ">>> yStepper command>>>"
        # ">>> Time cluster >>>"
        # ">>> Yaw >>>"
        # ">>> Stepper position >>>"
        # ">>> Encoders >>>"
        # ">>> Object detection >>>"
        # ">>> Ultrasonic Sensors Detect >>>"
        # ">>> Time cluster >>>"
        # ">>> Yaw >>>"
        # ">>> Stepper position >>>"
        # ">>> Encoders >>>"
        # ">>> Object detection >>>"
        # ">>> Ultrasonic Sensors Detect >>>"
      }
      frame True {
        # ">>State Logic Queue Reference >>"
        # ">>> Box Colour Detection >>>"
        # ">> Item Selection Bias >>"
        # ">>> IR Sensors >>>"
        # ">>> Line Sensor Cluster>>>"
        # ">>> Line Sensor Cluster>>>"
        # ">>> Motor control cluster >>>"
        # ">>> yStepper command>>>"
        # ">>> IR Sensors >>>"
        # ">>> Motor control cluster >>>"
        # ">>State Logic Queue Reference >>"
        # ">>Timeout>>"
        # ">>> yStepper command>>>"
        # ">>> Time cluster >>>"
        # ">>> Object detection >>>"
        # ">>> Yaw >>>"
        # ">>> Ultrasonic Sensors Detect >>>"
        # ">>> Encoders >>>"
        # ">>> Stepper position >>>"
        # ">>State Logic  >>"
        # ">>True Stop Next State >>"
        # ">>Action Queue>>"
        # ">> Manual override >>"
        # ">>> Time cluster >>>"
        # ">>> Yaw >>>"
        # ">>> Stepper position >>>"
        # ">>> Encoders >>>"
        # ">>> Object detection >>>"
        # ">>> Ultrasonic Sensors Detect >>>"
        # ">>Action Queue>>"
        # ">>State Logic Queue Reference >>"
        n191 = Or(x=w319, y=w320) -> (x .or. y?=w318:bool)
        n192 = Unbundle By Name(w299) -> ("Left IR Sensor"=w300:dbl, "Arm IR Sensor"=w296:dbl, "Bottom IR Sensor"=w291:dbl)
        n193 = Unbundle By Name(w294) -> ("Line Detected?"=w295:bool)
        n194 = Unbundle By Name(w305) -> ("Time up flag"=w306:bool)
        n195 = Unbundle By Name(w307) -> ("Yaw"=w308:dbl, "Compass"=w302:dbl)
        n196 = Unbundle By Name(w309) -> ("y Stepper Position"=w311:u8, "z Stepper Position"=w310:u8)
        n197 = Unbundle By Name(w325) -> ("xDistance"=w322:dbl, "yDistance"=w323:dbl, "wDistance"=w324:dbl)
        n198 = Unbundle By Name(w313) -> ("Recognized Object"=w312:bool, "Object X coordinate"=w315:dbl, "Object Y coordinate"=w314:dbl)
        n199 = Unbundle By Name(w336) -> ("PING_A"=w328:u8, "PING_B"=w327:u8, "PING_C"=w326:u8, "PING_D"=w321:u8)
        n200 = case shown="44" w335 {
          tunnel: [w341 w353 w367 w378 w496 w513 w559 w596 w651 w693 w741 w785 w840 w888 w932 w992 w1033 w1076 w1125 w1168 w1221 w1259 w1311 w1355 w1399 w1429 w1447 w1493 w1534 w1583 w1636 w1675 w1724 w1767 w1820 w1858 w1910 w1946 w1995 w2038 w2088 w2132 w2177 w2227 w2268 w2316 w2355 w2397 w2452 w2506 w2544 w2590 w2639 w2680 w2724 w2771 w2820 w2867 w2908] -> w334
          tunnel: w333 -> [w341 w356 w368 w381 w498 w514 w560 w605 w649 w697 w742 w791 w833 w891 w939 w982 w1036 w1082 w1124 w1171 w1211 w1265 w1301 w1350 w1390 w1429 w1437 w1496 w1540 w1582 w1635 w1681 w1723 w1770 w1810 w1864 w1900 w1950 w2002 w2043 w2093 w2137 w2181 w2225 w2269 w2317 w2357 w2407 w2462 w2505 w2548 w2596 w2638 w2684 w2728 w2775 w2827 w2872 w2918]
          tunnel: [State_Type_Definitions,_for_0.26g_versions_and_later_2."Idle" ("Enum") State_Type_Definitions,_for_0.26g_versions_and_later_2."Idle" ("Enum") w363 w380 State_Type_Definitions,_for_0.26g_versions_and_later_2."Shutdown" ("Enum") w515 w561 w603 w652 w694 w740 w786 w839 w889 w934 w991 w1034 w1083 w1126 w1170 w1220 w1266 w1310 w1356 w1391 State_Type_Definitions,_for_0.26g_versions_and_later_2."Idle" ("Enum") w1446 w1494 w1541 w1584 w1637 w1682 w1725 w1769 w1819 w1865 w1909 w1947 w1996 w2039 w2089 w2133 w2178 w2228 w2267 w2315 w2356 w2402 w2463 w2507 w2545 w2591 w2640 w2681 w2725 w2772 w2821 w2868 w2913] -> w332
          tunnel: w331 -> [_ _ w366 w384 _ w519 w566 w599 w648 w698 w749 w790 w837 w892 w938 w989 w1031 w1081 w1122 w1172 w1218 w1264 w1308 w1353 w1398 _ w1444 w1491 w1539 w1580 w1633 w1680 w1721 w1771 w1817 w1863 w1907 w1954 w2001 w2046 w2096 w2140 w2184 w2224 w2270 w2310 w2358 w2406 w2461 w2504 w2552 w2595 w2637 w2688 w2729 w2779 w2826 w2875 w2917]
          tunnel: w330 -> [_ _ _ w383 _ w518 w565 w598 w647 w699 w748 w789 w836 w885 w937 w988 w1030 w1080 w1121 w1173 w1217 w1263 w1307 w1352 w1396 _ w1443 w1490 w1538 w1579 w1632 w1679 w1720 w1772 w1816 w1862 w1906 w1949 w2000 w2045 w2095 w2139 w2180 w2223 w2271 w2311 w2359 w2405 w2460 w2503 w2551 w2594 w2636 w2687 w2730 w2774 w2825 w2874 w2916]
          tunnel: w329 -> [_ _ w365 w379 _ w517 w564 w597 w646 w700 w747 w788 w835 w884 w936 w990 w1032 w1079 w1120 w1174 w1219 w1262 w1309 w1351 w1397 _ w1445 w1492 w1537 w1578 w1631 w1678 w1719 w1773 w1818 w1861 w1908 w1953 w1999 w2044 w2094 w2138 w2183 w2222 w2272 w2312 w2360 w2404 w2459 w2502 w2550 w2593 w2635 w2686 w2731 w2778 w2824 w2873 w2915]
          tunnel: w318 -> [_ _ _ _ _ w504 w558 w604 w645 w701 w744 w784 w838 w890 w940 w983 w1037 w1077 w1123 w1175 w1212 w1260 w1302 w1354 w1394 _ w1438 w1497 w1535 w1581 w1634 w1676 w1722 w1774 w1811 w1859 w1901 w1952 w1994 w2042 w2092 w2136 w2182 w2221 w2273 w2313 w2361 w2403 w2458 w2501 w2549 w2592 w2634 w2685 w2732 w2777 w2819 w2871 w2914]
          tunnel: w328 -> [_ _ _ _ _ _ _ _ _ _ _ _ _ _ _ _ _ _ _ _ _ _ _ _ _ _ _ _ _ _ _ _ _ _ _ _ _ _ _ _ _ _ _ _ _ _ _ _ _ _ _ _ _ _ _ _ _ _ _]
          tunnel: w327 -> [_ _ _ _ _ _ _ _ w644 _ _ _ w829 w873 w930 _ _ _ _ _ _ _ _ _ _ _ _ w1483 _ _ _ _ _ _ _ _ _ _ _ _ _ _ _ _ _ _ _ _ w2456 _ _ _ _ _ _ _ _ _ _]
          tunnel: w326 -> [_ _ _ _ _ _ _ _ w643 _ _ _ w830 w874 w931 _ _ _ _ _ _ _ _ _ _ _ _ w1484 _ _ _ _ _ _ _ _ _ _ _ _ _ _ _ _ _ _ _ _ w2457 _ _ _ _ _ _ _ _ _ _]
          tunnel: w324 -> [_ _ _ _ _ _ _ _ _ _ w746 _ _ _ _ _ _ _ _ _ _ _ _ _ _ _ _ _ _ _ _ _ _ _ _ _ _ _ _ _ _ _ _ _ _ _ _ w2400 _ _ _ _ _ _ _ _ _ _ w2911]
          tunnel: w323 -> [_ _ _ _ _ w512 w557 _ _ w692 _ _ _ _ w935 _ _ _ _ _ _ _ _ _ _ _ _ _ _ _ _ _ _ _ _ _ _ _ _ _ _ _ _ _ _ _ _ _ w2448 _ _ _ _ _ _ _ _ _ _]
          tunnel: w322 -> [_ _ _ _ _ _ _ _ _ _ _ _ _ w879 _ _ _ _ _ _ _ _ _ _ _ _ _ _ _ _ w1622 _ _ _ _ _ _ _ _ _ _ _ _ _ w2262 _ _ _ _ _ _ _ w2633 _ _ _ _ _ _]
          tunnel: w321 -> [_ _ _ _ _ _ _ _ _ _ _ _ _ _ _ _ _ _ _ _ _ _ _ _ _ _ _ _ _ _ _ _ _ _ _ _ _ _ _ _ _ _ _ _ _ _ _ _ _ _ _ _ _ _ _ _ _ _ _]
          tunnel: [State_Type_Definitions,_for_0.26g_versions_and_later_2."Idle" ("Enum") State_Type_Definitions,_for_0.26g_versions_and_later_2."Idle" ("Enum") State_Type_Definitions,_for_0.26g_versions_and_later_2."Idle" ("Enum") State_Type_Definitions,_for_0.26g_versions_and_later_2."Idle" ("Enum") State_Type_Definitions,_for_0.26g_versions_and_later_2."Shutdown" ("Enum") w510 w555 w602 w650 w695 w737 w783 w832 w887 w933 w993 w1035 w1075 w1127 w1169 w1222 w1258 w1312 w1357 w1392 w1431 w1448 w1495 w1533 w1585 w1638 w1674 w1726 w1768 w1821 w1857 w1911 w1948 w1997 w2041 w2091 w2135 w2179 w2226 w2266 w2314 w2354 w2401 w2464 w2508 w2546 w2589 w2641 w2682 w2726 w2773 w2822 w2870 w2912] -> w317
          tunnel: w316 -> [_ _ w363 _ _ _ _ _ _ _ _ _ _ _ _ _ _ _ _ _ _ _ _ _ _ w1431 _ _ _ _ _ _ _ _ _ _ _ _ _ _ _ _ _ _ _ _ _ _ _ _ _ _ _ _ _ _ _ _ _]
          tunnel: w312 -> [_ _ _ _ _ _ _ _ _ _ _ _ _ _ _ _ _ _ _ _ _ _ _ _ w1393 _ _ _ _ _ _ _ _ _ _ _ _ _ _ _ _ _ _ _ _ _ _ _ _ _ _ _ _ _ _ _ _ _ _]
          tunnel: w315 -> [_ _ _ _ _ _ _ _ _ _ _ _ _ _ _ _ _ _ _ _ _ _ _ _ _ _ _ _ _ _ w1628 _ _ _ _ _ _ _ _ _ _ _ _ _ _ _ _ _ _ _ _ _ _ _ _ _ _ _ _]
          tunnel: w314 -> [_ _ _ _ _ _ _ _ _ _ _ _ _ _ _ _ _ _ _ w1164 _ _ _ _ _ _ _ _ _ _ _ _ _ w1763 _ _ _ _ _ _ _ _ _ _ _ _ _ _ _ _ _ _ _ _ _ _ _ _ _]
          tunnel: w311 -> [_ _ _ _ _ _ _ _ _ _ _ _ _ _ _ _ _ _ _ w1163 _ _ _ _ _ _ _ _ _ _ _ _ _ w1762 _ _ _ _ _ _ _ _ _ _ _ _ _ _ _ _ _ _ _ _ _ _ _ _ _]
          tunnel: w310 -> [_ _ _ _ _ _ _ w601 _ _ _ w781 _ _ _ w986 _ w1071 _ _ w1215 _ w1305 w1349 _ _ w1441 _ _ _ _ _ _ _ w1814 _ w1904 w1951 _ _ _ _ _ _ _ _ _ _ _ _ _ _ _ _ _ w2776 _ _ _]
          tunnel: w308 -> [_ _ _ _ _ _ _ _ _ _ _ _ _ _ _ _ _ _ _ _ _ _ _ _ _ _ _ _ _ _ _ _ _ _ _ _ _ _ _ _ _ _ _ _ _ _ _ _ _ _ _ _ _ _ _ _ _ _ _]
          tunnel: w306 -> [_ _ _ _ _ _ _ _ _ _ _ _ _ _ _ _ w1025 _ w1117 _ _ w1256 _ _ _ _ _ _ w1531 w1575 _ w1672 w1716 _ _ w1855 _ _ _ _ _ _ w2173 w2217 _ w2309 w2353 _ _ _ w2547 w2588 _ w2683 w2727 _ _ _ _]
          tunnel: w304 -> [w339 w351 w362 w376 w494 w509 w554 w600 w642 w696 w736 w782 w831 w883 w929 w981 w1028 w1074 w1118 w1166 w1210 w1257 w1300 w1346 w1389 w1432 w1436 w1488 w1532 w1576 w1629 w1673 w1717 w1765 w1809 w1856 w1899 w1945 w1998 w2040 w2090 w2134 w2176 w2220 w2275 w2319 w2363 w2409 w2466 w2510 w2554 w2598 w2646 w2690 w2734 w2770 w2823 w2869 w2920]
          tunnel: [w339 w350 w362 w376 w494 w509 w554 w600 w642 w696 w736 w782 w831 w883 w929 w981 w1028 w1074 w1118 w1165 w1210 w1257 w1300 w1346 w1389 w1432 w1436 w1488 w1532 w1576 w1629 w1673 w1717 w1764 w1809 w1856 w1899 w1945 w1998 w2040 w2090 w2134 w2176 w2220 w2275 w2319 w2363 w2409 w2466 w2510 w2554 w2598 w2646 w2690 w2734 w2770 w2823 w2869 w2920] -> w303
          tunnel: w302 -> [_ _ _ _ _ _ _ _ _ _ _ _ _ _ _ _ _ _ _ _ _ _ _ _ _ _ _ _ _ _ _ _ _ _ _ _ _ _ w1993 _ _ _ _ _ _ _ _ _ _ _ _ _ _ _ _ _ w2818 _ _]
          tunnel: [_ _ _ TRUE _ _ _ _ _ _ _ _ _ _ _ _ _ _ _ _ _ _ _ _ _ _ _ _ _ _ _ _ _ _ _ _ _ _ _ _ _ _ _ _ _ _ _ _ _ _ _ _ _ _ _ _ _ _ _] -> w301
          tunnel: w300 -> [_ _ _ _ _ _ _ _ _ _ _ _ _ _ _ _ _ _ _ _ _ _ _ _ _ _ _ _ _ _ _ _ _ _ _ _ _ _ _ _ _ _ _ _ _ _ _ _ _ _ _ _ _ _ _ _ _ _ _]
          tunnel: w298 -> [w338 w348 w361 w374 w493 w508 w553 w595 w641 w689 w735 w778 w824 w872 w928 w980 w1027 w1073 w1116 w1160 w1209 w1255 w1299 w1345 w1388 w1433 w1435 w1481 w1530 w1574 w1625 w1671 w1715 w1759 w1808 w1854 w1898 w1944 w1989 w2037 w2087 w2131 w2175 w2219 w2277 w2321 w2365 w2411 w2468 w2512 w2556 w2600 w2648 w2692 w2736 w2769 w2814 w2866 w2922]
          tunnel: [w338 w347 w361 w374 w493 w508 w553 w595 w641 w689 w735 w778 w824 w872 w928 w980 w1027 w1073 w1116 w1160 w1209 w1255 w1299 w1345 w1388 w1433 w1435 w1481 w1530 w1574 w1624 w1671 w1715 w1759 w1808 w1854 w1898 w1944 w1989 w2037 w2087 w2131 w2175 w2219 w2277 w2321 w2365 w2411 w2468 w2512 w2556 w2600 w2648 w2692 w2736 w2769 w2814 w2866 w2922] -> w297
          tunnel: w296 -> [_ _ _ _ _ _ _ _ _ _ _ _ _ _ _ _ _ _ _ _ _ _ _ _ _ _ _ _ _ _ _ _ _ _ _ _ _ _ _ _ w2085 _ _ _ _ _ _ _ w2454 _ _ _ _ _ _ _ _ _ _]
          tunnel: w295 -> [_ _ _ _ _ w505 _ _ _ _ _ _ _ _ w926 _ _ _ _ _ _ _ _ _ _ _ _ _ _ _ _ _ _ _ _ _ _ _ _ w2036 _ w2129 _ _ w2264 _ _ _ _ w2500 _ _ w2632 _ _ _ _ _ _]
          tunnel: [w337 w343 w360 w373 w492 w507 w552 w594 w640 w688 w734 w777 w823 w871 w927 w979 w1026 w1072 w1115 w1159 w1208 w1254 w1298 w1344 w1387 w1428 w1434 w1480 w1529 w1573 w1617 w1670 w1714 w1758 w1807 w1853 w1897 w1943 w1988 w2035 w2084 w2130 w2174 w2218 w2276 w2320 w2364 w2410 w2467 w2511 w2555 w2599 w2647 w2691 w2735 w2768 w2813 w2865 w2921] -> w293
          tunnel: w292 -> [w337 w343 w360 _ w492 w507 w552 w594 w640 w688 w734 w777 w823 w871 w927 w979 w1026 w1072 w1115 w1159 w1208 w1254 w1298 w1344 w1387 w1428 w1434 w1480 w1529 w1573 w1617 w1670 w1714 w1758 w1807 w1853 w1897 w1943 w1988 w2035 w2084 w2130 w2174 w2218 w2276 w2320 w2364 w2410 w2467 w2511 w2555 w2599 w2647 w2691 w2735 w2768 w2813 w2865 w2921]
          tunnel: w291 -> [_ _ _ _ _ _ _ _ _ _ _ _ _ _ _ _ _ _ _ _ _ _ _ _ _ _ _ _ _ _ _ _ _ _ _ _ _ _ _ _ w2083 _ _ _ _ _ _ _ _ _ _ _ _ _ _ _ _ w2862 _]
          tunnel: [_ _ _ _ _ _ _ _ w639 _ _ _ _ _ _ _ _ _ _ _ _ _ _ _ _ _ _ _ _ _ _ _ _ _ _ _ _ _ _ _ _ _ _ _ _ _ _ _ w2443 _ _ _ _ _ _ _ _ _ _] -> w290
          tunnel: [_ _ _ _ _ _ _ _ _ _ _ _ _ _ _ _ _ _ _ _ _ _ _ _ _ _ _ _ _ _ _ _ _ _ _ _ _ _ _ _ w2081 _ _ _ _ _ _ _ _ _ _ _ _ _ _ _ _ w2860 _] -> w289
          tunnel: [_ _ _ _ _ _ _ _ _ _ _ _ _ _ _ _ _ _ _ _ _ _ _ _ _ _ _ _ _ _ _ _ _ _ _ _ _ _ _ _ w2080 _ _ _ _ _ _ _ _ _ _ _ _ _ _ _ _ _ _] -> w288
          tunnel: w287 -> [_ _ _ _ _ _ _ _ _ _ _ _ _ _ _ _ _ _ _ _ _ _ _ _ _ _ _ _ _ _ _ _ _ _ _ _ _ _ _ _ _ _ _ _ _ _ _ _ _ _ _ _ _ _ _ _ _ _ _]
          frame 0 {
            # ">>> yStepper command>>>"
          }
          frame 1 {
            # ">>> yStepper command>>>"
            n201 = for {
              shift-right: [w359] -> w353
              shift-left: w356 -> [w358]
              tunnel: string[] ["INIT", "RESET ARM", "RESET FLAGS", "RESET YAW", "NAVX CALIBRATE"] -> [w357] mode=indexing
              n202 = Enqueue Element(queue=w358, element=w357) -> (queue out=w359:refnum<queue>)  [unwired: 2 in, 2 out]
            }
            n203 = Bundle By Name(cluster=w351, "yStepper desired"=u8 0) -> (w350:T20)
            n204 = Bundle By Name(cluster=w348, "ySpeed"=0.0, "xSpeed"=0.0, "wSpeed"=0.0) -> (w347:T19)
          }
          frame 3 {
            # ">>Action Queue>>"
            # ">>> Motor control cluster >>>"
            # ">>> yStepper command>>>"
            n205 = Flush Queue(queue=w366, error in (no error)=w365) -> ()  [unwired: 3 out]